vi "s.vi"() -> ()   [LabVIEW 2013]
uses:
  <vilib>/regexp/Match Regular Expression.xnode
panel:
  out "Numeric":dbl
  in  "Tab Control 25":enum32{"Page 1", "Page 2"}(tab)
  in  "edit":bool
  out "Table Control":string[][](table)
  in  "String":string
  in  "flag 8":u16(ring) items=["Admin", "User"]
  in  "String":string
  in  "String":string
  in  "delete":bool
  in  "add":bool
  out "channel":dbl
  out "URL":string="C:\\Users\\kiat\\Downloads\\asd.mp4"
  in  "Tab Control 24":enum32{"Page 1", "Page 2"}(tab)
  in  "WindowsMediaPlayer":refnum<k7>(container)
  in  "backward":bool
  in  "foward":bool
  in  "pause":bool
  in  "stop":bool
  in  "flag 7":u16(ring) items=["1", "2", "3"]
  in  "play":bool
  in  "?":dbl(slide) scale=0.0..100.0
  in  "Tab Control 23":enum32{"Page 1", "Page 2"}(tab)
  in  "?":bool
  in  "String":string
  in  "?":bool
  in  "?":dbl(slide) scale=16.0..27.0
  in  "Tab Control 22":enum32{"Page 1", "Page 2"}(tab)
  in  "?":bool
  in  "String":string
  in  "?":bool
  in  "?":dbl(slide) scale=16.0..27.0
  in  "Tab Control 21":enum32{"Page 1", "Page 2"}(tab)
  in  "?":bool
  in  "String":string
  in  "?":bool
  in  "?":dbl(slide) scale=16.0..27.0
  in  "Tab Control 19":enum32{"Page 1", "Page 2"}(tab)
  in  "?":bool
  in  "?":bool
  in  "?":bool
  in  "Tab Control 18":enum32{"Page 1", "Page 2"}(tab)
  in  "?":bool
  in  "start hour 3":u16(ring) items=["1", "2", "3", "4", "5", "6", "7", "8", "9", "10", "11", "12"]
  in  "flag 6":u16(ring) items=["AM", "PM"]
  in  "start min 3":u16(ring) items=["0", "1", "2", "3", "4", "5", "6", "7", "8", "9", "10", "11", "12", "13", "14", "15", "16", "17", "18", "19", "20", "21", "22", "23", "24", "25", "26", "27", "28", "29", "30", "31", "32", "33", "34", "35", "36", "37", "38", "39", "40", "41", "42", "43", "44", "45", "46", "47", "48", "49", "50", "51", "52", "53", "54", "55", "56", "57", "58", "59"]
  in  "end hour 3":u16(ring) items=["1", "2", "3", "4", "5", "6", "7", "8", "9", "10", "11", "12"]
  in  "end min 3":u16(ring) items=["0", "1", "2", "3", "4", "5", "6", "7", "8", "9", "10", "11", "12", "13", "14", "15", "16", "17", "18", "19", "20", "21", "22", "23", "24", "25", "26", "27", "28", "29", "30", "31", "32", "33", "34", "35", "36", "37", "38", "39", "40", "41", "42", "43", "44", "45", "46", "47", "48", "49", "50", "51", "52", "53", "54", "55", "56", "57", "58", "59"]
  in  "flag 5":u16(ring) items=["AM", "PM"]
  in  "String":string
  in  "?":bool
  in  "?":dbl(slide) scale=0.0..4.0
  in  "Tab Control 17":enum32{"Page 1", "Page 2"}(tab)
  in  "flag 3":u16(ring) items=["AM", "PM"]
  in  "end min 2":u16(ring) items=["0", "1", "2", "3", "4", "5", "6", "7", "8", "9", "10", "11", "12", "13", "14", "15", "16", "17", "18", "19", "20", "21", "22", "23", "24", "25", "26", "27", "28", "29", "30", "31", "32", "33", "34", "35", "36", "37", "38", "39", "40", "41", "42", "43", "44", "45", "46", "47", "48", "49", "50", "51", "52", "53", "54", "55", "56", "57", "58", "59"]
  in  "end hour 2":u16(ring) items=["1", "2", "3", "4", "5", "6", "7", "8", "9", "10", "11", "12"]
  in  "start min 2":u16(ring) items=["0", "1", "2", "3", "4", "5", "6", "7", "8", "9", "10", "11", "12", "13", "14", "15", "16", "17", "18", "19", "20", "21", "22", "23", "24", "25", "26", "27", "28", "29", "30", "31", "32", "33", "34", "35", "36", "37", "38", "39", "40", "41", "42", "43", "44", "45", "46", "47", "48", "49", "50", "51", "52", "53", "54", "55", "56", "57", "58", "59"]
  in  "flag 4":u16(ring) items=["AM", "PM"]
  in  "start hour 2":u16(ring) items=["1", "2", "3", "4", "5", "6", "7", "8", "9", "10", "11", "12"]
  in  "?":bool
  in  "String":string
  in  "?":bool
  in  "?":dbl(slide) scale=0.0..4.0
  in  "Tab Control 16":enum32{"Page 1", "Page 2"}(tab)
  in  "?":bool
  in  "?":bool
  in  "?":bool
  in  "Tab Control 15":enum32{"Page 1", "Page 2"}(tab)
  in  "OK Button 32":bool
  in  "OK Button 31":bool
  in  "?":bool
  in  "Tab Control 14":enum32{"Page 1", "Page 2"}(tab)
  in  "OK Button 27":bool
  in  "OK Button 26":bool
  in  "OK Button 25":bool
  in  "?":bool
  in  "Tab Control 13":enum32{"Page 1", "Page 2"}(tab)
  in  "OK Button 24":bool
  in  "OK Button 23":bool
  in  "OK Button 22":bool
  in  "OK Button 21":bool
  in  "OK Button 20":bool
  in  "OK Button 19":bool
  in  "?":bool
  in  "Tab Control 12":enum32{"Page 1", "Page 2"}(tab)
  in  "?":bool
  in  "?":bool
  in  "?":bool
  in  "Tab Control 11":enum32{"Page 1", "Page 2"}(tab)
  in  "flag":u16(ring) items=["AM", "PM"]
  in  "end min 1":u16(ring) items=["0", "1", "2", "3", "4", "5", "6", "7", "8", "9", "10", "11", "12", "13", "14", "15", "16", "17", "18", "19", "20", "21", "22", "23", "24", "25", "26", "27", "28", "29", "30", "31", "32", "33", "34", "35", "36", "37", "38", "39", "40", "41", "42", "43", "44", "45", "46", "47", "48", "49", "50", "51", "52", "53", "54", "55", "56", "57", "58", "59"]
  in  "end hour 1":u16(ring) items=["1", "2", "3", "4", "5", "6", "7", "8", "9", "10", "11", "12"]
  in  "start min 1":u16(ring) items=["0", "1", "2", "3", "4", "5", "6", "7", "8", "9", "10", "11", "12", "13", "14", "15", "16", "17", "18", "19", "20", "21", "22", "23", "24", "25", "26", "27", "28", "29", "30", "31", "32", "33", "34", "35", "36", "37", "38", "39", "40", "41", "42", "43", "44", "45", "46", "47", "48", "49", "50", "51", "52", "53", "54", "55", "56", "57", "58", "59"]
  in  "flag 2":u16(ring) items=["AM", "PM"]
  in  "start hour 1":u16(ring) items=["1", "2", "3", "4", "5", "6", "7", "8", "9", "10", "11", "12"]
  in  "?":bool
  in  "String":string
  in  "?":bool
  in  "?":dbl(slide) scale=0.0..4.0
  in  "Tab Control 10":enum32{"Page 1", "Page 2"}(tab)
  in  "Tab Control 9":enum32{"Page 1", "Page 2"}(tab)
  in  "OK Button 18":bool
  in  "?":bool
  in  "Tab Control 8":enum32{"Page 1", "Page 2"}(tab)
  in  "OK Button 17":bool
  in  "?":bool
  in  "Tab Control 7":enum32{"Page 1", "Page 2"}(tab)
  in  "OK Button 16":bool
  in  "?":bool
  in  "Tab Control 6":enum32{"Page 1", "Page 2"}(tab)
  in  "OK Button 15":bool
  in  "?":bool
  in  "Tab Control 5":enum32{"Page 1", "Page 2"}(tab)
  in  "OK Button 14":bool
  in  "OK Button 13":bool
  in  "OK Button 12":bool
  in  "OK Button 11":bool
  in  "?":bool
  in  "Tab Control 4":enum32{"Page 1", "Page 2"}(tab)
  in  "OK Button 10":bool
  in  "OK Button 9":bool
  in  "OK Button 8":bool
  in  "OK Button 7":bool
  in  "OK Button 6":bool
  in  "OK Button 5":bool
  in  "?":bool
  in  "stop":bool
  in  "OK Button 3":bool
  in  "Tab Control 3":enum32{"Page 1", "Page 2"}(tab)
  in  "?":bool
  in  "?":bool
  in  "?":bool
  in  "?":bool
  in  "?":bool
  in  "?":bool
  in  "Tab Control 2":enum32{"Page 1"}(tab)
  in  "?":bool
  in  "?":bool
  in  "?":bool
  in  "?":bool
  in  "?":bool
  in  "?":bool
  in  "Tab Control":enum32{"Page 1", "Page 2"}(tab)
  in  "String 2":string caption="String"
  in  "OK Button":bool
  in  "String":string
  # "Master room \nlight 1"
  # "Master room \ndoor 1"
  # "Master room \nldoor 1"
  # "Open Area \nlight 1"
  # "Garrden \nlight 1"
  # "Living room \nlight 1"
  # "Living room \nlight 1"
  # "Master bathroom \nlight 1"
  # "Master room \nlight 1"
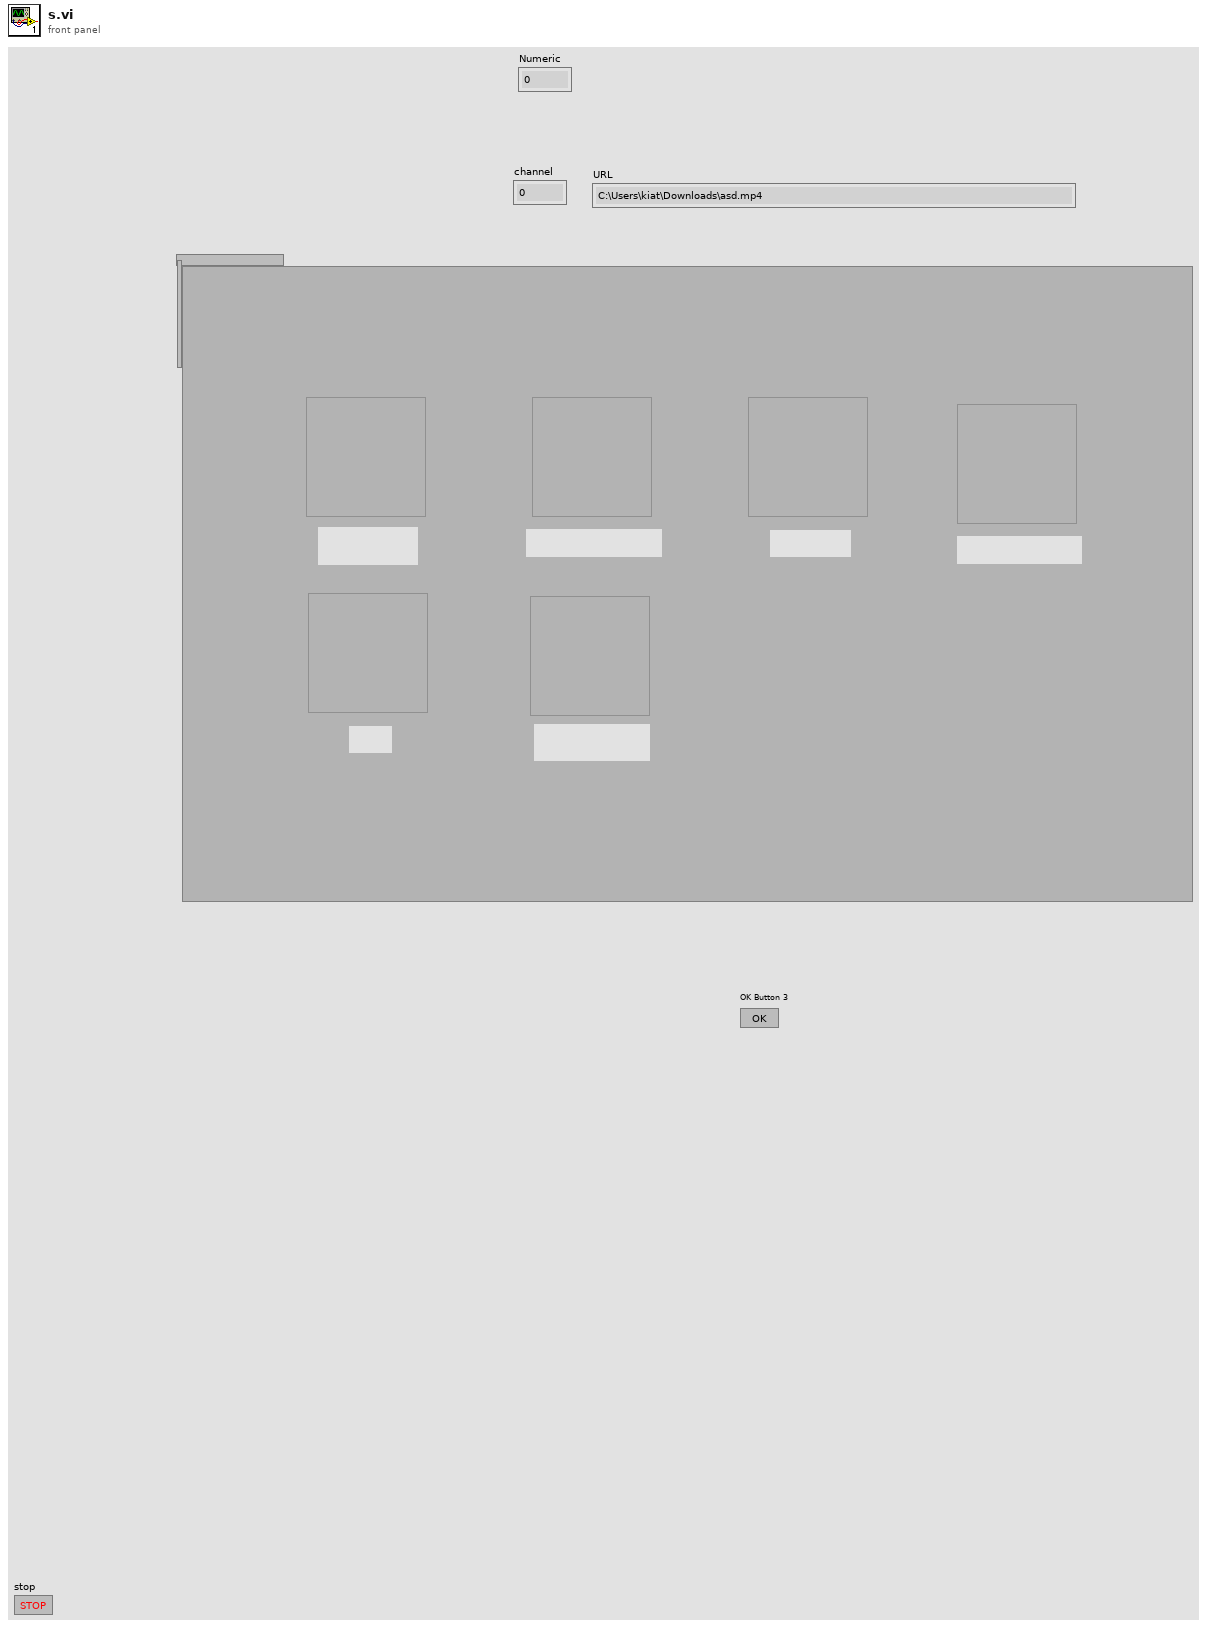
[diagram p1: front panel]
types:
  T1 = enum8{"Enabled", "Disabled", "Disabled and Grayed Out"}
  T2 = enum16{"open", "replace", "create", "open or create", "replace or create", "replace or create with confirmation"}
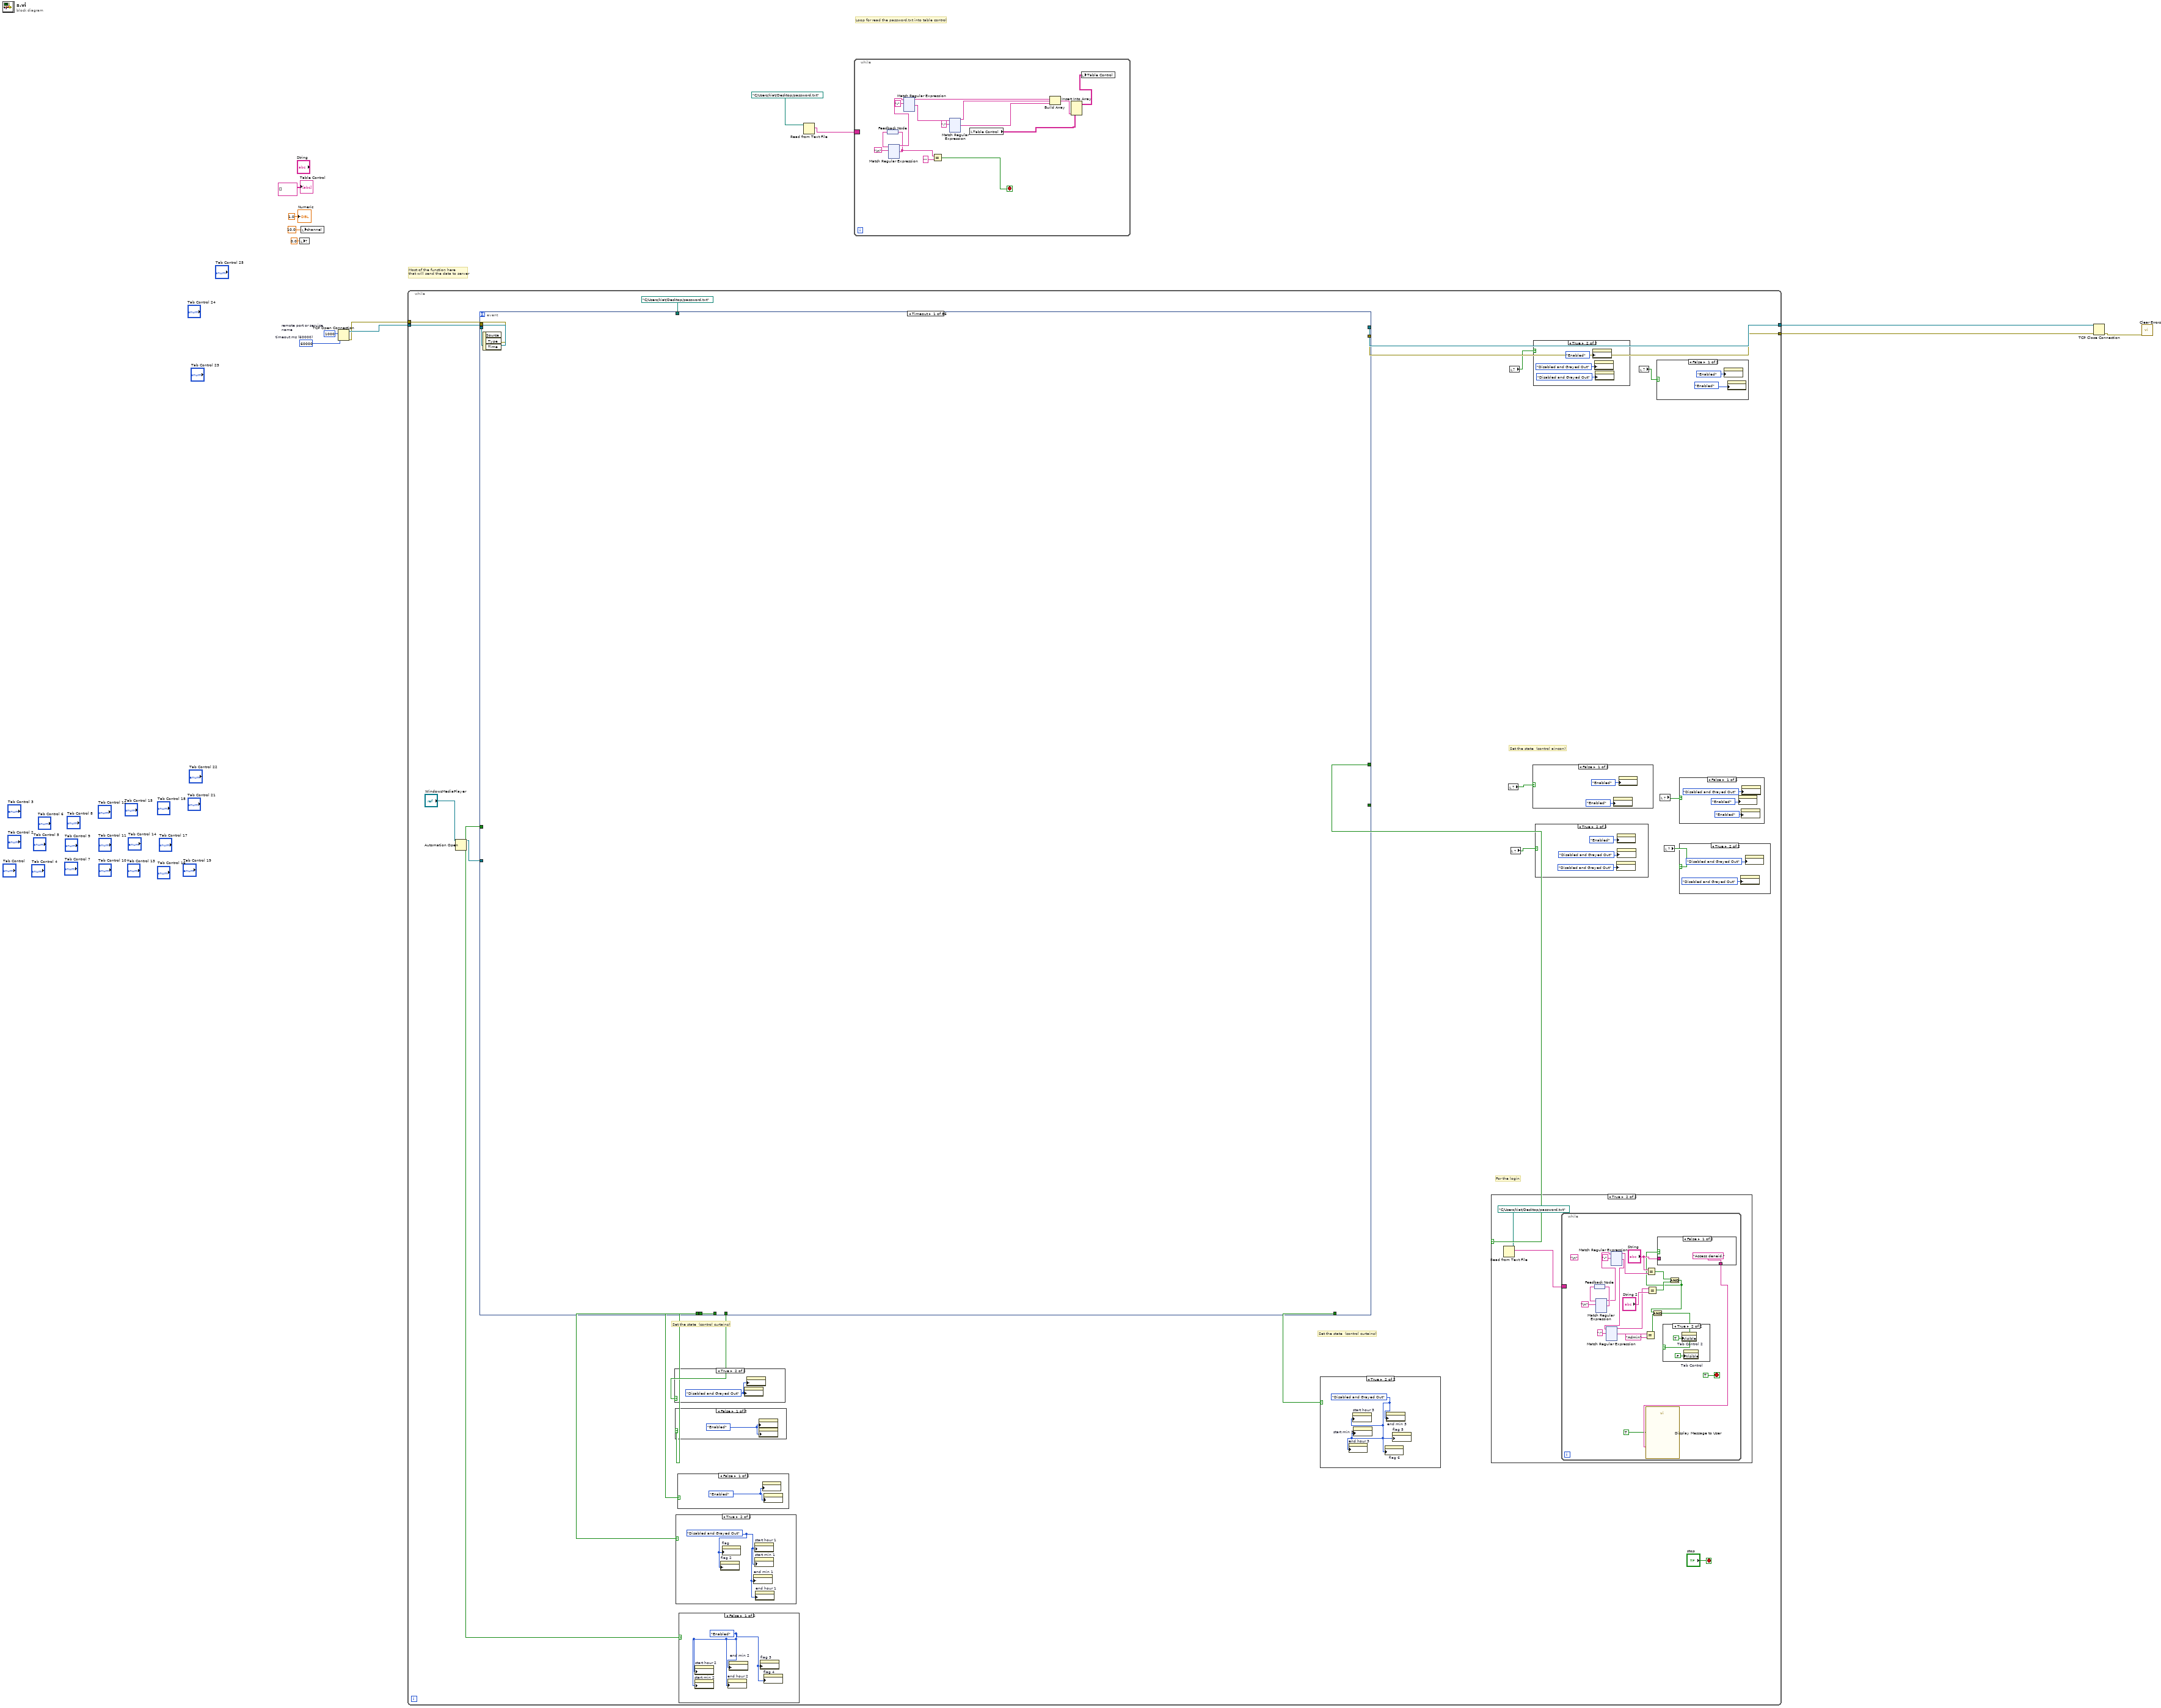
[diagram p0: block diagram]
diagram:
  w12 = 60000  # timeout ms (60000)
  w13 = u16 1000  # remote port or service name
  # "Most of the function here\nthat will send the data to server"
  # "Loop for read the password.txt into table control"
  n1 = local write item#?(0.0) -> ()
  n2 = local write "channel"(10.0 ("Numeric 2")) -> ()
  n3 = TCP Open Connection(remote port or service name=w13, timeout ms (60000)=w12) -> (connection ID=w9:refnum<k5>, error out=w8:errorcluster)  [unwired: 3 in]
  n4 = while {
    tunnel: w9 -> [w33]
    tunnel: w8 -> [w32]
    tunnel: [w30] -> w10
    tunnel: [w29] -> w7
    stop <- "stop" stop-if-true
    # "Set the state  (control air-con)"
    # "Set the state  (control curtains)"
    # "Set the state  (control curtains)"
    # "For the login"
    n5 = Automation Open(Automation Refnum="WindowsMediaPlayer") -> (Automation Refnum=w15:refnum<k7>)  [unwired: 3 in, 1 out]
    n6 = event shown="[0] Timeout" {
      selector: _ -> [_ _ _ _ _ _ _ _ _ _ _ _ _ _ _ _ _ _ _ _ _ _ _ _ _ _ _ _ _ _ _ _ _ _ _ _ _ _ _ _ _ _ _ _ _ _ _ _ _ _ _ _ _ _ _ _ _ _ _ _ _ _ _ _ _ _ _ _ _ _ _ _ _ _ _ _ _ _ _ _ _ _ _ _ _ _]
      dyn-events: _ -> [_ _ _ _ _ _ _ _ _ _ _ _ _ _ _ _ _ _ _ _ _ _ _ _ _ _ _ _ _ _ _ _ _ _ _ _ _ _ _ _ _ _ _ _ _ _ _ _ _ _ _ _ _ _ _ _ _ _ _ _ _ _ _ _ _ _ _ _ _ _ _ _ _ _ _ _ _ _ _ _ _ _ _ _ _ _]
      timeout: _ -> [_ _ _ _ _ _ _ _ _ _ _ _ _ _ _ _ _ _ _ _ _ _ _ _ _ _ _ _ _ _ _ _ _ _ _ _ _ _ _ _ _ _ _ _ _ _ _ _ _ _ _ _ _ _ _ _ _ _ _ _ _ _ _ _ _ _ _ _ _ _ _ _ _ _ _ _ _ _ _ _ _ _ _ _ _ _]
      tunnel: [_ "OK Button" _ _ _ _ _ _ _ _ _ _ _ _ _ _ _ _ _ _ _ _ _ _ _ _ _ _ _ _ _ _ _ _ _ _ _ _ _ _ _ _ _ _ _ _ _ _ _ _ _ _ _ _ _ _ _ _ _ _ _ _ _ _ _ _ _ _ _ _ _ _ _ _ _ _ _ _ _ _ _ _ _ _ _ _] -> w34
      tunnel: w33 -> [_ _ _ _ w498 w510 _ _ w568 w577 _ w615 w630 w645 w655 w667 _ w700 w715 w728 _ w765 _ _ w821 _ _ w879 w890 w902 w916 _ _ _ _ w1015 w1026 w1043 _ w1080 _ w1123 w1138 w1150 _ _ _ w2585 _ w2622 w2636 w2650 _ w2687 w2697 w2709 w2721 w2734 w2746 w2759 w2770 w2784 w2797 w2805 w2816 w2831 w2843 _ w2874 w2887 w2900 w2912 w2922 w2933 w2947 w2975 w3005 w3035 _ w3065 _ _ w3123 w3133 w3145 w3158]
      tunnel: [_ _ _ _ w504 w516 _ _ w571 w585 _ w617 w629 w643 w661 w673 _ w708 w720 w729 _ w763 _ _ w822 _ _ w883 w891 w901 w918 _ _ _ _ w1017 w1029 w1040 _ w1078 _ w1121 w1136 w1153 _ _ _ w2583 _ w2620 w2635 w2653 _ w2692 w2705 w2712 w2728 w2739 w2753 w2764 w2776 w2788 w2795 w2811 w2824 w2836 w2848 _ w2880 w2892 w2904 w2916 w2928 w2943 w2951 w2977 w3006 w3036 _ w3069 _ _ w3127 w3139 w3150 w3161] -> w30
      tunnel: w32 -> [_ _ _ _ w499 w511 _ _ w569 w580 _ w614 w631 w644 w656 w668 _ w703 w712 w727 _ w764 _ _ w820 _ _ w878 w889 w903 w915 _ _ _ _ w1014 w1027 w1042 _ w1079 _ w1122 w1137 w1151 _ _ _ w2584 _ w2621 w2637 w2651 _ w2684 w2696 w2710 w2722 w2735 w2747 w2758 w2769 w2783 w2796 w2804 w2819 w2830 w2840 _ w2875 w2888 w2897 w2909 w2921 w2932 w2948 w2974 w3004 w3034 _ w3066 _ _ w3120 w3132 w3144 w3157]
      tunnel: [_ _ _ _ w503 w515 _ _ w572 w584 _ w616 w628 w642 w660 w672 _ w707 w719 w730 _ w762 _ _ w823 _ _ w882 w892 w900 w917 _ _ _ _ w1016 w1028 w1039 _ w1077 _ w1120 w1135 w1152 _ _ _ w2582 _ w2619 w2634 w2652 _ w2691 w2704 w2711 w2729 w2740 w2752 w2763 w2775 w2787 w2794 w2810 w2823 w2835 w2847 _ w2879 w2891 w2905 w2917 w2929 w2942 w2950 w2978 w3007 w3037 _ w3070 _ _ w3128 w3140 w3151 w3162] -> w29
      tunnel: [_ _ _ _ _ _ _ _ _ _ _ _ _ _ _ _ _ _ _ _ _ _ _ _ _ _ _ _ _ _ "?" _ _ _ _ _ _ _ _ _ _ _ _ _ _ _ _ _ _ _ _ _ _ _ _ _ _ _ _ _ _ _ _ _ _ _ _ _ _ _ _ _ _ _ _ _ _ _ _ _ _ _ _ _ _ _] -> w28
      tunnel: [_ _ _ _ _ _ _ _ _ _ _ _ _ _ _ _ _ _ _ _ _ _ _ _ "?" _ _ _ _ _ _ _ _ _ _ _ _ _ _ _ _ _ _ _ _ _ _ _ _ _ _ _ _ _ _ _ _ _ _ _ _ _ _ _ _ _ _ _ _ _ _ _ _ _ _ _ _ _ _ _ _ _ _ _ _ _] -> w27
      tunnel: [_ _ _ _ _ _ _ _ _ _ _ _ _ _ _ _ _ _ _ "?" _ _ _ _ _ _ _ _ _ _ _ _ _ _ _ _ _ _ _ _ _ _ _ _ _ _ _ _ _ _ _ _ _ _ _ _ _ _ _ _ _ _ _ _ _ _ _ _ _ _ _ _ _ _ _ _ _ _ _ _ _ _ _ _ _ _] -> w26
      tunnel: [_ _ _ _ _ _ _ _ _ _ _ _ _ _ _ _ _ _ _ _ _ _ _ _ _ _ _ _ _ _ _ _ _ _ _ _ _ _ _ _ _ _ _ _ _ _ _ _ _ _ _ _ _ _ _ _ _ _ _ _ _ _ _ _ _ _ _ _ _ _ _ _ _ _ _ "?" _ _ _ _ _ _ _ _ _ _] -> w25
      tunnel: [_ _ _ _ _ _ _ _ _ _ _ _ _ _ _ _ _ _ _ _ _ _ _ _ _ _ _ _ _ _ _ _ _ _ _ _ _ _ _ _ _ _ _ _ _ _ _ _ _ _ _ _ _ _ _ _ _ _ _ _ _ _ _ _ _ _ _ _ _ _ _ _ _ _ _ _ "?" _ _ _ _ _ _ _ _ _] -> w24
      tunnel: [_ _ _ _ _ _ _ _ _ _ _ _ _ _ _ _ _ _ _ _ _ _ _ _ _ _ _ _ _ _ _ _ _ _ _ _ _ _ _ _ _ _ _ _ _ _ _ _ _ _ _ _ _ _ _ _ _ _ _ _ _ _ _ _ _ _ _ _ _ _ _ _ _ _ _ _ _ "?" _ _ _ _ _ _ _ _] -> w23
      tunnel: [_ _ _ _ _ _ _ _ _ _ _ _ w626 _ _ _ _ _ _ _ _ _ _ _ _ _ _ _ _ _ _ _ _ _ _ _ _ _ _ _ _ _ _ _ _ _ _ _ _ _ _ _ _ _ _ _ _ _ _ _ _ _ _ _ _ _ _ _ _ _ _ _ _ _ _ _ _ _ _ _ _ _ _ _ _ _] -> _
      tunnel: w15 -> [_ _ _ _ _ _ _ _ _ _ _ _ _ _ _ _ _ _ _ _ _ _ _ _ _ _ _ _ _ _ _ _ _ _ _ _ _ _ _ w1081 _ w1132 w1147 w1162 _ _ _ w2593 _ w2631 _ _ _ _ _ _ _ _ _ _ _ _ _ _ _ _ _ _ _ _ _ _ _ _ _ _ _ _ _ _ _ _ _ _ _ _]
      tunnel: path "C:/Users/kiat/Desktop/password.txt" ("file (use dialog)") -> [_ _ _ _ _ _ _ _ _ _ _ _ _ _ _ _ _ _ _ _ _ _ _ _ _ _ _ _ _ _ _ _ _ _ _ _ _ _ _ _ _ _ _ _ w1166 w1440 w2196 _ _ _ _ _ _ _ _ _ _ _ _ _ _ _ _ _ _ _ _ _ _ _ _ _ _ _ _ _ _ _ _ _ _ _ _ _ _ _]
      event Timeout {
        n7 = event-data() -> ()  [unwired: 1 in, 3 out]
      }
      event "OK Button": Value Change {
        n8 = event-data() -> ()  [unwired: 1 in, 6 out]
      }
      event "OK Button 3": Value Change {
        n9 = event-data() -> ()  [unwired: 1 in, 6 out]
        n10 = property on="Tab Control 5" class="TabCtl (strict)"("Visible"=FALSE) -> ()  [unwired: 2 in, 2 out]
        n11 = property on="Tab Control 3" class="TabCtl (strict)"("Visible"=FALSE) -> ()  [unwired: 2 in, 2 out]
        n12 = property on="Tab Control 21" class="TabCtl (strict)"("Visible"=FALSE) -> ()  [unwired: 2 in, 2 out]
        n13 = property on="Tab Control 9" class="TabCtl (strict)"("Visible"=FALSE) -> ()  [unwired: 2 in, 2 out]
        n14 = property on="Tab Control 22" class="TabCtl (strict)"("Visible"=FALSE) -> ()  [unwired: 2 in, 2 out]
        n15 = property on="Tab Control 23" class="TabCtl (strict)"("Visible"=FALSE) -> ()  [unwired: 2 in, 2 out]
        n16 = property on="Tab Control 4" class="TabCtl (strict)"("Visible"=FALSE) -> ()  [unwired: 2 in, 2 out]
        n17 = property on="Tab Control 12" class="TabCtl (strict)"("Visible"=FALSE) -> ()  [unwired: 2 in, 2 out]
        n18 = property on="Tab Control 19" class="TabCtl (strict)"("Visible"=FALSE) -> ()  [unwired: 2 in, 2 out]
        n19 = property on="Tab Control 24" class="TabCtl (strict)"("Visible"=FALSE) -> ()  [unwired: 2 in, 2 out]
        n20 = property on="Tab Control 7" class="TabCtl (strict)"("Visible"=FALSE) -> ()  [unwired: 2 in, 2 out]
        n21 = property on="Tab Control 14" class="TabCtl (strict)"("Visible"=FALSE) -> ()  [unwired: 2 in, 2 out]
        n22 = property on="Tab Control 16" class="TabCtl (strict)"("Visible"=FALSE) -> ()  [unwired: 2 in, 2 out]
        n23 = property on="Tab Control 13" class="TabCtl (strict)"("Visible"=FALSE) -> ()  [unwired: 2 in, 2 out]
        n24 = property on="Tab Control 25" class="TabCtl (strict)"("Visible"=FALSE) -> ()  [unwired: 2 in, 2 out]
        n25 = property on="Tab Control 15" class="TabCtl (strict)"("Visible"=FALSE) -> ()  [unwired: 2 in, 2 out]
        n26 = property on="Tab Control 8" class="TabCtl (strict)"("Visible"=FALSE) -> ()  [unwired: 2 in, 2 out]
        n27 = property on="Tab Control 10" class="TabCtl (strict)"("Visible"=FALSE) -> ()  [unwired: 2 in, 2 out]
        n28 = property on="Tab Control 6" class="TabCtl (strict)"("Visible"=FALSE) -> ()  [unwired: 2 in, 2 out]
        n29 = property on="Tab Control 11" class="TabCtl (strict)"("Visible"=FALSE) -> ()  [unwired: 2 in, 2 out]
        n30 = property on="Tab Control 2" class="TabCtl (strict)"("Visible"=FALSE) -> ()  [unwired: 2 in, 2 out]
        n31 = property on="Tab Control 18" class="TabCtl (strict)"("Visible"=FALSE) -> ()  [unwired: 2 in, 2 out]
        n32 = property on="Tab Control 17" class="TabCtl (strict)"("Visible"=FALSE) -> ()  [unwired: 2 in, 2 out]
        n33 = property on="Tab Control" class="TabCtl (strict)"("Visible"=TRUE) -> ()  [unwired: 2 in, 2 out]
      }
      event Value Change {
        n34 = event-data() -> ()  [unwired: 1 in, 6 out]
        n35 = property on="Tab Control 17" class="TabCtl (strict)"("Visible"=FALSE) -> ()  [unwired: 2 in, 2 out]
        n36 = property on="Tab Control 3" class="TabCtl (strict)"("Visible"=FALSE) -> ()  [unwired: 2 in, 2 out]
        n37 = property on="Tab Control 11" class="TabCtl (strict)"("Visible"=FALSE) -> ()  [unwired: 2 in, 2 out]
        n38 = property on="Tab Control 6" class="TabCtl (strict)"("Visible"=TRUE) -> ()  [unwired: 2 in, 2 out]
        n39 = property on="Tab Control 10" class="TabCtl (strict)"("Visible"=FALSE) -> ()  [unwired: 2 in, 2 out]
        n40 = property on="Tab Control 18" class="TabCtl (strict)"("Visible"=FALSE) -> ()  [unwired: 2 in, 2 out]
        n41 = property on="Tab Control 2" class="TabCtl (strict)"("Visible"=FALSE) -> ()  [unwired: 2 in, 2 out]
        n42 = property on="Tab Control 5" class="TabCtl (strict)"("Visible"=FALSE) -> ()  [unwired: 2 in, 2 out]
        n43 = property on="Tab Control 9" class="TabCtl (strict)"("Visible"=FALSE) -> ()  [unwired: 2 in, 2 out]
        n44 = property on="Tab Control" class="TabCtl (strict)"("Visible"=FALSE) -> ()  [unwired: 2 in, 2 out]
        n45 = property on="Tab Control 8" class="TabCtl (strict)"("Visible"=FALSE) -> ()  [unwired: 2 in, 2 out]
        n46 = property on="Tab Control 22" class="TabCtl (strict)"("Visible"=FALSE) -> ()  [unwired: 2 in, 2 out]
        n47 = property on="Tab Control 12" class="TabCtl (strict)"("Visible"=FALSE) -> ()  [unwired: 2 in, 2 out]
        n48 = property on="Tab Control 4" class="TabCtl (strict)"("Visible"=FALSE) -> ()  [unwired: 2 in, 2 out]
        n49 = property on="Tab Control 23" class="TabCtl (strict)"("Visible"=FALSE) -> ()  [unwired: 2 in, 2 out]
        n50 = property on="Tab Control 19" class="TabCtl (strict)"("Visible"=FALSE) -> ()  [unwired: 2 in, 2 out]
        n51 = property on="Tab Control 7" class="TabCtl (strict)"("Visible"=FALSE) -> ()  [unwired: 2 in, 2 out]
        n52 = property on="Tab Control 14" class="TabCtl (strict)"("Visible"=FALSE) -> ()  [unwired: 2 in, 2 out]
        n53 = property on="Tab Control 13" class="TabCtl (strict)"("Visible"=FALSE) -> ()  [unwired: 2 in, 2 out]
        n54 = property on="Tab Control 15" class="TabCtl (strict)"("Visible"=FALSE) -> ()  [unwired: 2 in, 2 out]
        n55 = property on="Tab Control 24" class="TabCtl (strict)"("Visible"=FALSE) -> ()  [unwired: 2 in, 2 out]
        n56 = property on="Tab Control 21" class="TabCtl (strict)"("Visible"=FALSE) -> ()  [unwired: 2 in, 2 out]
        n57 = property on="Tab Control 16" class="TabCtl (strict)"("Visible"=FALSE) -> ()  [unwired: 2 in, 2 out]
      }
      event Value Change {
        n58 = event-data() -> ()  [unwired: 1 in, 6 out]
        n59 = Type Cast(x=0.0) -> (*(type *) &x=w501:string)  [unwired: 1 in]
        n60 = TCP Write(connection ID=w498, data in=w501, error in (no error)=w499) -> (connection ID out=w497:refnum<k5>, error out=w496:errorcluster)  [unwired: 1 in, 1 out]
        n61 = Bundle("?", 13.0) -> (w502:cluster{bool, dbl})  [unwired: 1 in]
        n62 = Type Cast(x=w502) -> (*(type *) &x=w507:string)  [unwired: 1 in]
        n63 = TCP Write(connection ID=w497, data in=w507, error in (no error)=w496) -> (connection ID out=w504:refnum<k5>, error out=w503:errorcluster)  [unwired: 1 in, 1 out]
      }
      event "OK Button 15": Value Change {
        n64 = event-data() -> ()  [unwired: 1 in, 6 out]
        n65 = Type Cast(x=0.0) -> (*(type *) &x=w513:string)  [unwired: 1 in]
        n66 = TCP Write(connection ID=w510, data in=w513, error in (no error)=w511) -> (connection ID out=w509:refnum<k5>, error out=w508:errorcluster)  [unwired: 1 in, 1 out]
        n67 = Bundle("OK Button 15"="OK Button 15", 12.0) -> (w517:cluster{"OK Button 15":bool, dbl})  [unwired: 1 in]
        n68 = Type Cast(x=w517) -> (*(type *) &x=w519:string)  [unwired: 1 in]
        n69 = TCP Write(connection ID=w509, data in=w519, error in (no error)=w508) -> (connection ID out=w516:refnum<k5>, error out=w515:errorcluster)  [unwired: 1 in, 1 out]
      }
      event Value Change {
        n70 = event-data() -> ()  [unwired: 1 in, 6 out]
        n71 = property on="Tab Control 18" class="TabCtl (strict)"("Visible"=FALSE) -> ()  [unwired: 2 in, 2 out]
        n72 = property on="Tab Control 17" class="TabCtl (strict)"("Visible"=FALSE) -> ()  [unwired: 2 in, 2 out]
        n73 = property on="Tab Control 21" class="TabCtl (strict)"("Visible"=FALSE) -> ()  [unwired: 2 in, 2 out]
        n74 = property on="Tab Control 16" class="TabCtl (strict)"("Visible"=FALSE) -> ()  [unwired: 2 in, 2 out]
        n75 = property on="Tab Control 10" class="TabCtl (strict)"("Visible"=FALSE) -> ()  [unwired: 2 in, 2 out]
        n76 = property on="Tab Control 5" class="TabCtl (strict)"("Visible"=FALSE) -> ()  [unwired: 2 in, 2 out]
        n77 = property on="Tab Control 3" class="TabCtl (strict)"("Visible"=FALSE) -> ()  [unwired: 2 in, 2 out]
        n78 = property on="Tab Control 6" class="TabCtl (strict)"("Visible"=FALSE) -> ()  [unwired: 2 in, 2 out]
        n79 = property on="Tab Control 23" class="TabCtl (strict)"("Visible"=FALSE) -> ()  [unwired: 2 in, 2 out]
        n80 = property on="Tab Control 12" class="TabCtl (strict)"("Visible"=FALSE) -> ()  [unwired: 2 in, 2 out]
        n81 = property on="Tab Control 2" class="TabCtl (strict)"("Visible"=FALSE) -> ()  [unwired: 2 in, 2 out]
        n82 = property on="Tab Control 7" class="TabCtl (strict)"("Visible"=TRUE) -> ()  [unwired: 2 in, 2 out]
        n83 = property on="Tab Control 4" class="TabCtl (strict)"("Visible"=FALSE) -> ()  [unwired: 2 in, 2 out]
        n84 = property on="Tab Control 24" class="TabCtl (strict)"("Visible"=FALSE) -> ()  [unwired: 2 in, 2 out]
        n85 = property on="Tab Control 11" class="TabCtl (strict)"("Visible"=FALSE) -> ()  [unwired: 2 in, 2 out]
        n86 = property on="Tab Control" class="TabCtl (strict)"("Visible"=FALSE) -> ()  [unwired: 2 in, 2 out]
        n87 = property on="Tab Control 8" class="TabCtl (strict)"("Visible"=FALSE) -> ()  [unwired: 2 in, 2 out]
        n88 = property on="Tab Control 9" class="TabCtl (strict)"("Visible"=FALSE) -> ()  [unwired: 2 in, 2 out]
        n89 = property on="Tab Control 22" class="TabCtl (strict)"("Visible"=FALSE) -> ()  [unwired: 2 in, 2 out]
        n90 = property on="Tab Control 14" class="TabCtl (strict)"("Visible"=FALSE) -> ()  [unwired: 2 in, 2 out]
        n91 = property on="Tab Control 13" class="TabCtl (strict)"("Visible"=FALSE) -> ()  [unwired: 2 in, 2 out]
        n92 = property on="Tab Control 15" class="TabCtl (strict)"("Visible"=FALSE) -> ()  [unwired: 2 in, 2 out]
        n93 = property on="Tab Control 19" class="TabCtl (strict)"("Visible"=FALSE) -> ()  [unwired: 2 in, 2 out]
      }
      event Value Change {
        n94 = event-data() -> ()  [unwired: 1 in, 6 out]
        n95 = property on="Tab Control 16" class="TabCtl (strict)"("Visible"=FALSE) -> ()  [unwired: 2 in, 2 out]
        n96 = property on="Tab Control 6" class="TabCtl (strict)"("Visible"=FALSE) -> ()  [unwired: 2 in, 2 out]
        n97 = property on="Tab Control 10" class="TabCtl (strict)"("Visible"=FALSE) -> ()  [unwired: 2 in, 2 out]
        n98 = property on="Tab Control 18" class="TabCtl (strict)"("Visible"=FALSE) -> ()  [unwired: 2 in, 2 out]
        n99 = property on="Tab Control 17" class="TabCtl (strict)"("Visible"=FALSE) -> ()  [unwired: 2 in, 2 out]
        n100 = property on="Tab Control 21" class="TabCtl (strict)"("Visible"=FALSE) -> ()  [unwired: 2 in, 2 out]
        n101 = property on="Tab Control 5" class="TabCtl (strict)"("Visible"=FALSE) -> ()  [unwired: 2 in, 2 out]
        n102 = property on="Tab Control 4" class="TabCtl (strict)"("Visible"=FALSE) -> ()  [unwired: 2 in, 2 out]
        n103 = property on="Tab Control 3" class="TabCtl (strict)"("Visible"=FALSE) -> ()  [unwired: 2 in, 2 out]
        n104 = property on="Tab Control" class="TabCtl (strict)"("Visible"=FALSE) -> ()  [unwired: 2 in, 2 out]
        n105 = property on="Tab Control 2" class="TabCtl (strict)"("Visible"=FALSE) -> ()  [unwired: 2 in, 2 out]
        n106 = property on="Tab Control 12" class="TabCtl (strict)"("Visible"=FALSE) -> ()  [unwired: 2 in, 2 out]
        n107 = property on="Tab Control 22" class="TabCtl (strict)"("Visible"=FALSE) -> ()  [unwired: 2 in, 2 out]
        n108 = property on="Tab Control 7" class="TabCtl (strict)"("Visible"=FALSE) -> ()  [unwired: 2 in, 2 out]
        n109 = property on="Tab Control 11" class="TabCtl (strict)"("Visible"=FALSE) -> ()  [unwired: 2 in, 2 out]
        n110 = property on="Tab Control 8" class="TabCtl (strict)"("Visible"=TRUE) -> ()  [unwired: 2 in, 2 out]
        n111 = property on="Tab Control 9" class="TabCtl (strict)"("Visible"=FALSE) -> ()  [unwired: 2 in, 2 out]
        n112 = property on="Tab Control 14" class="TabCtl (strict)"("Visible"=FALSE) -> ()  [unwired: 2 in, 2 out]
        n113 = property on="Tab Control 13" class="TabCtl (strict)"("Visible"=FALSE) -> ()  [unwired: 2 in, 2 out]
        n114 = property on="Tab Control 15" class="TabCtl (strict)"("Visible"=FALSE) -> ()  [unwired: 2 in, 2 out]
        n115 = property on="Tab Control 24" class="TabCtl (strict)"("Visible"=FALSE) -> ()  [unwired: 2 in, 2 out]
        n116 = property on="Tab Control 23" class="TabCtl (strict)"("Visible"=FALSE) -> ()  [unwired: 2 in, 2 out]
        n117 = property on="Tab Control 19" class="TabCtl (strict)"("Visible"=FALSE) -> ()  [unwired: 2 in, 2 out]
      }
      event Value Change {
        n118 = event-data() -> ()  [unwired: 1 in, 6 out]
        n119 = Type Cast(x=0.0) -> ()  [unwired: 1 in, 1 out]
        n120 = TCP Write(connection ID=w568, error in (no error)=w569) -> (connection ID out=w567:refnum<k5>, error out=w566:errorcluster)  [unwired: 2 in, 1 out]
        n121 = Bundle("?", 17.0) -> (w574:cluster{bool, dbl})  [unwired: 1 in]
        n122 = Type Cast(x=w574) -> (*(type *) &x=w576:string)  [unwired: 1 in]
        n123 = TCP Write(connection ID=w567, data in=w576, error in (no error)=w566) -> (connection ID out=w571:refnum<k5>, error out=w572:errorcluster)  [unwired: 1 in, 1 out]
      }
      event "OK Button 17": Value Change {
        n124 = event-data() -> ()  [unwired: 1 in, 6 out]
        n125 = Type Cast(x=0.0) -> (*(type *) &x=w582:string)  [unwired: 1 in]
        n126 = TCP Write(connection ID=w577, data in=w582, error in (no error)=w580) -> (connection ID out=w578:refnum<k5>, error out=w579:errorcluster)  [unwired: 1 in, 1 out]
        n127 = Bundle("OK Button 17"="OK Button 17", 18.0) -> (w586:cluster{"OK Button 17":bool, dbl})  [unwired: 1 in]
        n128 = Type Cast(x=w586) -> (*(type *) &x=w588:string)  [unwired: 1 in]
        n129 = TCP Write(connection ID=w578, data in=w588, error in (no error)=w579) -> (connection ID out=w585:refnum<k5>, error out=w584:errorcluster)  [unwired: 1 in, 1 out]
      }
      event Value Change {
        n130 = event-data() -> ()  [unwired: 1 in, 6 out]
        n131 = property on="Tab Control 6" class="TabCtl (strict)"("Visible"=FALSE) -> ()  [unwired: 2 in, 2 out]
        n132 = property on="Tab Control 18" class="TabCtl (strict)"("Visible"=FALSE) -> (error out=w594:errorcluster)  [unwired: 2 in, 1 out]
        n133 = property on="Tab Control 17" class="TabCtl (strict)"("Visible"=FALSE) -> ()  [unwired: 2 in, 2 out]
        n134 = property on="Tab Control 21" class="TabCtl (strict)"("Visible"=FALSE) -> ()  [unwired: 2 in, 2 out]
        n135 = property on="Tab Control 10" class="TabCtl (strict)"("Visible"=FALSE) -> ()  [unwired: 2 in, 2 out]
        n136 = property on="Tab Control 12" class="TabCtl (strict)"(error in=w594, "Visible"=FALSE) -> ()  [unwired: 1 in, 2 out]
        n137 = property on="Tab Control 24" class="TabCtl (strict)"("Visible"=FALSE) -> ()  [unwired: 2 in, 2 out]
        n138 = property on="Tab Control 5" class="TabCtl (strict)"("Visible"=FALSE) -> ()  [unwired: 2 in, 2 out]
        n139 = property on="Tab Control 4" class="TabCtl (strict)"("Visible"=FALSE) -> ()  [unwired: 2 in, 2 out]
        n140 = property on="Tab Control 3" class="TabCtl (strict)"("Visible"=FALSE) -> ()  [unwired: 2 in, 2 out]
        n141 = property on="Tab Control" class="TabCtl (strict)"("Visible"=FALSE) -> ()  [unwired: 2 in, 2 out]
        n142 = property on="Tab Control 2" class="TabCtl (strict)"("Visible"=FALSE) -> ()  [unwired: 2 in, 2 out]
        n143 = property on="Tab Control 22" class="TabCtl (strict)"("Visible"=FALSE) -> ()  [unwired: 2 in, 2 out]
        n144 = property on="Tab Control 7" class="TabCtl (strict)"("Visible"=FALSE) -> ()  [unwired: 2 in, 2 out]
        n145 = property on="Tab Control 9" class="TabCtl (strict)"("Visible"=TRUE) -> ()  [unwired: 2 in, 2 out]
        n146 = property on="Tab Control 11" class="TabCtl (strict)"("Visible"=FALSE) -> ()  [unwired: 2 in, 2 out]
        n147 = property on="Tab Control 8" class="TabCtl (strict)"("Visible"=FALSE) -> ()  [unwired: 2 in, 2 out]
        n148 = property on="Tab Control 16" class="TabCtl (strict)"("Visible"=FALSE) -> ()  [unwired: 2 in, 2 out]
        n149 = property on="Tab Control 23" class="TabCtl (strict)"("Visible"=FALSE) -> ()  [unwired: 2 in, 2 out]
        n150 = property on="Tab Control 14" class="TabCtl (strict)"("Visible"=FALSE) -> ()  [unwired: 2 in, 2 out]
        n151 = property on="Tab Control 13" class="TabCtl (strict)"("Visible"=FALSE) -> ()  [unwired: 2 in, 2 out]
        n152 = property on="Tab Control 15" class="TabCtl (strict)"("Visible"=FALSE) -> ()  [unwired: 2 in, 2 out]
        n153 = property on="Tab Control 19" class="TabCtl (strict)"("Visible"=FALSE) -> ()  [unwired: 2 in, 2 out]
      }
      event Value Change {
        # "Air conditional - Bed room (slider)"
        n154 = event-data() -> ()  [unwired: 1 in, 6 out]
        n155 = Type Cast(x=5.0) -> (*(type *) &x=w619:string)  [unwired: 1 in]
        n156 = TCP Write(connection ID=w615, data in=w619, error in (no error)=w614) -> (connection ID out=w621:refnum<k5>, error out=w622:errorcluster)  [unwired: 1 in, 1 out]
        n157 = Bundle("?", "?", 1.0) -> (w623:cluster{bool, dbl, dbl})  [unwired: 1 in]
        n158 = Type Cast(x=w623) -> (*(type *) &x=w625:string)  [unwired: 1 in]
        n159 = TCP Write(connection ID=w621, data in=w625, error in (no error)=w622) -> (connection ID out=w617:refnum<k5>, error out=w616:errorcluster)  [unwired: 1 in, 1 out]
      }
      event Value Change {
        # "Air conditional - Bed room"
        n160 = event-data() -> ()  [unwired: 1 in, 6 out]
        n161 = local read item#9() -> (w626:bool)
        n162 = local read item#12() -> (w627:dbl)
        n163 = Type Cast(x=5.0) -> (*(type *) &x=w632:string)  [unwired: 1 in]
        n164 = TCP Write(connection ID=w630, data in=w632, error in (no error)=w631) -> (connection ID out=w634:refnum<k5>, error out=w635:errorcluster)  [unwired: 1 in, 1 out]
        n165 = Bundle(w626, w627, 1.0) -> (w636:cluster{bool, dbl, dbl})  [unwired: 1 in]
        n166 = Type Cast(x=w636) -> (*(type *) &x=w638:string)  [unwired: 1 in]
        n167 = TCP Write(connection ID=w634, data in=w638, error in (no error)=w635) -> (connection ID out=w629:refnum<k5>, error out=w628:errorcluster)  [unwired: 1 in, 1 out]
      }
      event Value Change {
        # "Air conditional - Bed room (set temperature)"
        n168 = event-data() -> ()  [unwired: 1 in, 6 out]
        n169 = Decimal String To Number(string="String") -> (number=w640:i32)  [unwired: 2 in, 1 out]
        n170 = Type Cast(x=6.0) -> (*(type *) &x=w646:string)  [unwired: 1 in]
        n171 = TCP Write(connection ID=w645, data in=w646, error in (no error)=w644) -> (connection ID out=w648:refnum<k5>, error out=w649:errorcluster)  [unwired: 1 in, 1 out]
        n172 = Bundle("?", w640, 1.0) -> (w650:cluster{bool, i32, dbl})  [unwired: 1 in]
        n173 = Type Cast(x=w650) -> (*(type *) &x=w652:string)  [unwired: 1 in]
        n174 = TCP Write(connection ID=w648, data in=w652, error in (no error)=w649) -> (connection ID out=w643:refnum<k5>, error out=w642:errorcluster)  [unwired: 1 in, 1 out]
      }
      event Value Change {
        n175 = event-data() -> ()  [unwired: 1 in, 6 out]
        n176 = Type Cast(x=0.0) -> (*(type *) &x=w658:string)  [unwired: 1 in]
        n177 = TCP Write(connection ID=w655, data in=w658, error in (no error)=w656) -> (connection ID out=w654:refnum<k5>, error out=w653:errorcluster)  [unwired: 1 in, 1 out]
        n178 = Bundle("?", 15.0) -> (w662:cluster{bool, dbl})  [unwired: 1 in]
        n179 = Type Cast(x=w662) -> (*(type *) &x=w664:string)  [unwired: 1 in]
        n180 = TCP Write(connection ID=w654, data in=w664, error in (no error)=w653) -> (connection ID out=w661:refnum<k5>, error out=w660:errorcluster)  [unwired: 1 in, 1 out]